vi "Dresden R2R Sputter 03.02.2018 IY24.vi"() -> ()   [LabVIEW 2009] (continued)
                        n624 = local read "Ch3_Bp_bv_open_L_safety"() -> (w1488)
                        n625 = case shown="False" w1488 {
                          frame #0 {
                            n626 = local write "Error Message"(data[5B] ("Error Message")) -> ()
                          }
                          frame #1 {
                            n627 = local write "Ch3_4_4_do"(T/1 ("Ch3_Do_Bp_bv_L")) -> ()
                          }
                        }
                      }
                    }
                    n628 = case shown="True" w1483 {
                      frame #0 {
                      }
                      frame #1 {
                        n629 = local read "Ch3_Bp_bv_close_L_safety"() -> (w1485)
                        n630 = case shown="False" w1485 {
                          frame #0 {
                            n631 = local write "Error Message"(data[5B] ("Error Message")) -> ()
                          }
                          frame #1 {
                            n632 = local write "Ch3_4_4_do"(i16? 0 ("Ch3_Do_Bp_bv_L")) -> ()
                          }
                        }
                      }
                    }
                  }
                }
                n633 = stacked-sequence {
                  frame #0 {
                    n634 = Or(x="Bp_bv_open_ch1_R_gui", y="Bp_bv_open_ch1_R") -> (x .or. y?=w1532)
                    n635 = Or(x="Bp_bv_close_ch1_R_gui", y="Bp_bv_close_ch1_R") -> (x .or. y?=w1531)
                    n636 = case shown="True" w1531 {
                      frame #0 {
                      }
                      frame #1 {
                        n637 = local read "Ch1_Bp_bv_close_R_safety"() -> (w1533)
                        n638 = case shown="True" w1533 {
                          frame #0 {
                            n639 = local write "Error Message"("BP-BV can not be opened.\nReason: SP does not work \nwhen system is under vacuum. \nIf system is  not under vacuum, TP-BV \nor PL-VBV  can be  open,or \nMP can work." ("Error Message")) -> ()
                          }
                          frame #1 {
                          }
                        }
                      }
                    }
                    n640 = case shown="True" w1532 {
                      frame #0 {
                      }
                      frame #1 {
                        n641 = local read "Ch1_Bp_bv_open_R_safety"() -> (w1535)
                        n642 = case shown="True" w1535 {
                          frame #0 {
                            n643 = local write "Error Message"("BP-BV can not be opened.\nReason: SP does not work \nwhen system is under vacuum. \nIf system is  not under vacuum, TP-BV \nor PL-VBV  can be  open,or \nMP can work." ("Error Message")) -> ()
                          }
                          frame #1 {
                          }
                        }
                      }
                    }
                  }
                }
                n644 = stacked-sequence {
                  frame #0 {
                    n645 = Or(x="Bp_bv_close_ch4_L_gui", y="Bp_bv_close_ch4_L") -> (x .or. y?=w1472)
                    n646 = Or(x="Bp_bv_open_ch4_L_gui", y="Bp_bv_open_ch4_L") -> (x .or. y?=w1467)
                    n647 = case shown="True" w1467 {
                      frame #0 {
                      }
                      frame #1 {
                        n648 = local read "Ch4_Bp_bv_open_L_safety"() -> (w1476)
                        n649 = case shown="True" w1476 {
                          frame #0 {
                            n650 = local write "Error Message"("BP-BV can not be opened.\nReason: SP does not work \nwhen system is under vacuum. \nIf system is  not under vacuum, TP-BV \nor PL-VBV  can be  open,or \nMP can work." ("Error Message")) -> ()
                          }
                          frame #1 {
                            n651 = local write "Ch4_4_4_do"(T/1 ("Ch3_Do_Bp_bv_L")) -> ()
                          }
                        }
                      }
                    }
                    n652 = case shown="True" w1472 {
                      frame #0 {
                      }
                      frame #1 {
                        n653 = local read "Ch4_Bp_bv_close_L_safety"() -> (w1473)
                        n654 = case shown="True" w1473 {
                          frame #0 {
                            n655 = local write "Error Message"("BP-BV can not be opened.\nReason: SP does not work \nwhen system is under vacuum. \nIf system is  not under vacuum, TP-BV \nor PL-VBV  can be  open,or \nMP can work." ("Error Message")) -> ()
                          }
                          frame #1 {
                            n656 = local write "Ch4_4_4_do"(i16? 0 ("Ch3_Do_Bp_bv_L")) -> ()
                          }
                        }
                      }
                    }
                  }
                }
                n657 = stacked-sequence {
                  frame #0 {
                    n658 = Or(x="Bp_bv_open_ch2_R_gui", y="Bp_bv_open_ch2_R") -> (x .or. y?=w1519)
                    n659 = Or(x="Bp_bv_close_ch2_R_gui", y="Bp_bv_close_ch2_R") -> (x .or. y?=w1520)
                    n660 = case shown="True" w1519 {
                      frame #0 {
                      }
                      frame #1 {
                        n661 = local read "Ch2_Bp_bv_open_R_safety"() -> (w1524)
                        n662 = case shown="True" w1524 {
                          frame #0 {
                            n663 = local write "Error Message"("BP-BV can not be opened.\nReason: SP does not work \nwhen system is under vacuum. \nIf system is  not under vacuum, TP-BV \nor PL-VBV  can be  open,or \nMP can work." ("Error Message")) -> ()
                          }
                          frame #1 {
                            n664 = local write "Ch2_4_3_do"(T/1 ("Ch1_Do_Bp_bv_R")) -> ()
                          }
                        }
                      }
                    }
                    n665 = case shown="True" w1520 {
                      frame #0 {
                      }
                      frame #1 {
                        n666 = local read "Ch2_Bp_bv_close_R_safety"() -> (w1521)
                        n667 = case shown="True" w1521 {
                          frame #0 {
                            n668 = local write "Error Message"("BP-BV can not be opened.\nReason: SP does not work \nwhen system is under vacuum. \nIf system is  not under vacuum, TP-BV \nor PL-VBV  can be  open,or \nMP can work." ("Error Message")) -> ()
                          }
                          frame #1 {
                            n669 = local write "Ch2_4_3_do"(i16? 0 ("Ch1_Do_Bp_bv_R")) -> ()
                          }
                        }
                      }
                    }
                  }
                }
                n670 = stacked-sequence {
                  frame #0 {
                    n671 = Or(x="Bp_bv_open_ch3_R_gui", y="Bp_bv_open_ch3_R") -> (x .or. y?=w1503)
                    n672 = Or(x="Bp_bv_close_ch3_R_gui", y="Bp_bv_close_ch3_R") -> (x .or. y?=w1506)
                    n673 = case shown="True" w1503 {
                      frame #0 {
                      }
                      frame #1 {
                        n674 = local read "Ch3_Bp_bv_open_R_safety"() -> (w1512)
                        n675 = case shown="True" w1512 {
                          frame #0 {
                            n676 = local write "Error Message"("BP-BV can not be opened.\nReason: SP does not work \nwhen system is under vacuum. \nIf system is  not under vacuum, TP-BV \nor PL-VBV  can be  open,or \nMP can work." ("Error Message")) -> ()
                          }
                          frame #1 {
                            n677 = local write "Ch3_4_3_do"(T/1 ("Ch1_Do_Bp_bv_R")) -> ()
                          }
                        }
                      }
                    }
                    n678 = case shown="True" w1506 {
                      frame #0 {
                      }
                      frame #1 {
                        n679 = local read "Ch3_Bp_bv_close_R_safety"() -> (w1509)
                        n680 = case shown="True" w1509 {
                          frame #0 {
                            n681 = local write "Error Message"("BP-BV can not be opened.\nReason: SP does not work \nwhen system is under vacuum. \nIf system is  not under vacuum, TP-BV \nor PL-VBV  can be  open,or \nMP can work." ("Error Message")) -> ()
                          }
                          frame #1 {
                            n682 = local write "Ch3_4_3_do"(i16? 0 ("Ch1_Do_Bp_bv_R")) -> ()
                          }
                        }
                      }
                    }
                  }
                }
                n683 = stacked-sequence {
                  frame #0 {
                    n684 = Or(x="Bp_bv_open_ch2_L_gui", y="Bp_bv_open_ch2_L_tab") -> (x .or. y?=w1494)
                    n685 = Or(x="Bp_bv_close_ch2_L_gui", y="Bp_bv_close_ch2_L") -> (x .or. y?=w1491)
                    n686 = case shown="True" w1494 {
                      frame #0 {
                      }
                      frame #1 {
                        n687 = local read "Ch2_Bp_bv_open_L_safety"() -> (w1500)
                        n688 = case shown="False" w1500 {
                          frame #0 {
                            n689 = local write "Error Message"("BP-BV can not be opened.\nReason: SP does not work \nwhen system is under vacuum. \nIf system is  not under vacuum, TP-BV \nor PL-VBV  can be  open,or \nMP can work." ("Error Message")) -> ()
                          }
                          frame #1 {
                            n690 = local write "Ch2_4_4_do"(T/1 ("Ch1_Do_Bp_bv_R")) -> ()
                          }
                        }
                      }
                    }
                    n691 = case shown="True" w1491 {
                      frame #0 {
                      }
                      frame #1 {
                        n692 = local read "Ch2_Bp_bv_close_L_safety"() -> (w1497)
                        n693 = case shown="False" w1497 {
                          frame #0 {
                            n694 = local write "Error Message"("BP-BV can not be opened.\nReason: SP does not work \nwhen system is under vacuum. \nIf system is  not under vacuum, TP-BV \nor PL-VBV  can be  open,or \nMP can work." ("Error Message")) -> ()
                          }
                          frame #1 {
                            n695 = local write "Ch2_4_4_do"(i16? 0 ("Ch1_Do_Bp_bv_R")) -> ()
                          }
                        }
                      }
                    }
                  }
                }
              }
              frame #1 {
              }
            }
          }
        }
        n696 = stacked-sequence {
          frame #0 {
            n697 = Or(x="Ch1_Ch_vbv_open_gui", y="Ch1_Ch_vbv_open") -> (x .or. y?=w1542)
            n698 = Or(x="Ch1_Ch_vbv_close_gui", y="Ch1_Ch_vbv_close") -> (x .or. y?=w1541)
            n699 = case shown="True" w1542 {
              frame #0 {
              }
              frame #1 {
                n700 = local read "Ch1_Ch_vbv_open_safety"() -> (w1562)
                n701 = case shown="False" w1562 {
                  frame #0 {
                    n702 = local write "Error Message"("CH-VBV can not be opened.\nReason : * TP-BV can be open.     \n *Tp can not be stopped.\n*CH-CC can be open.    \n*BG-BV can be open.     " ("Error Message")) -> ()
                  }
                  frame #1 {
                    n703 = stacked-sequence {
                      frame #0 {
                        n704 = local write "Ch1_Ch_atm_do"(i16? 0 ("Ch1_Ch_vbv_do")) -> ()
                      }
                      frame #1 {
                        n705 = Wait (ms)(milliseconds to wait=i32? 500) -> ()  [unwired: 1 out]
                      }
                      frame #2 {
                        n706 = local write "Ch1_Ch_vbv_do"(T/1 ("Ch1_Ch_vbv_do")) -> ()
                      }
                      frame #3 {
                        n707 = Wait (ms)(milliseconds to wait=i32? 500) -> ()  [unwired: 1 out]
                      }
                    }
                  }
                }
              }
            }
            n708 = case shown="True" w1541 {
              frame #0 {
              }
              frame #1 {
                n709 = local write "Ch1_Ch_vbv_do"(i16? 0 ("Ch1_Ch_vbv_do")) -> ()
              }
            }
            n710 = Or(x="Ch2_Ch_vbv_open_gui", y="Ch2_Ch_vbv_open") -> (x .or. y?=w1559)
            n711 = Or(x="Ch2_Ch_vbv_close", y="Ch2_Ch_vbv_close_gui") -> (x .or. y?=w1560)
            n712 = case shown="True" w1559 {
              frame #0 {
              }
              frame #1 {
                n713 = local read "Ch2_Ch_vbv_open_safety"() -> (w1583)
                n714 = case shown="False" w1583 {
                  frame #0 {
                    n715 = local write "Error Message"("CH-VBV can not be opened.\nReason : * TP-BV can be open.     \n *Tp can not be stopped.\n*CH-CC can be open.    \n*BG-BV can be open.     " ("Error Message")) -> ()
                  }
                  frame #1 {
                    n716 = stacked-sequence {
                      frame #0 {
                        n717 = local write "Ch2_Ch_atm_do"(i16? 0 ("Ch1_Ch_vbv_do")) -> ()
                      }
                      frame #1 {
                        n718 = Wait (ms)(milliseconds to wait=i32? 500) -> ()  [unwired: 1 out]
                      }
                      frame #2 {
                        n719 = local write "Ch2_Ch_vbv_do"(T/1 ("Ch1_Ch_vbv_do")) -> ()
                      }
                      frame #3 {
                        n720 = Wait (ms)(milliseconds to wait=i32? 500) -> ()  [unwired: 1 out]
                      }
                    }
                  }
                }
              }
            }
            n721 = case shown="False" w1560 {
              frame #0 {
              }
              frame #1 {
                n722 = local write "Ch2_Ch_vbv_do"(i16? 0 ("Ch1_Ch_vbv_do")) -> ()
              }
            }
            n723 = Or(x="Ch3_Ch_vbv_open_gui", y="Ch3_Ch_vbv_open") -> (x .or. y?=w1558)
            n724 = Or(x="Ch3_Ch_vbv_close_gui", y="Ch3_Ch_vbv_close") -> (x .or. y?=w1557)
            n725 = case shown="True" w1558 {
              frame #0 {
              }
              frame #1 {
                n726 = local read "Ch3_Ch_vbv_open_safety"() -> (w1576)
                n727 = case shown="True" w1576 {
                  frame #0 {
                    n728 = local write "Error Message"("CH-VBV can not be opened.\nReason : * TP-BV can be open.     \n *Tp can not be stopped.\n*CH-CC can be open.    \n*BG-BV can be open.     " ("Error Message")) -> ()
                  }
                  frame #1 {
                    n729 = stacked-sequence {
                      frame #0 {
                        n730 = local write "Ch3_Ch_atm_do"(i16? 0 ("Ch1_Ch_vbv_do")) -> ()
                      }
                      frame #1 {
                        n731 = Wait (ms)(milliseconds to wait=i32? 500) -> ()  [unwired: 1 out]
                      }
                      frame #2 {
                        n732 = local write "Ch3_Ch_vbv_do"(T/1 ("Ch1_Ch_vbv_do")) -> ()
                      }
                      frame #3 {
                        n733 = Wait (ms)(milliseconds to wait=i32? 500) -> ()  [unwired: 1 out]
                      }
                    }
                  }
                }
              }
            }
            n734 = case shown="True" w1557 {
              frame #0 {
              }
              frame #1 {
                n735 = local write "Ch3_Ch_vbv_do"(i16? 0 ("Ch1_Ch_vbv_do")) -> ()
              }
            }
            n736 = Or(x="Ch4_Ch_vbv_open_gui", y="Ch4_Ch_vbv_open") -> (x .or. y?=w1556)
            n737 = Or(x="Ch4_Ch_vbv_close_gui", y="Ch4_Ch_vbv_close") -> (x .or. y?=w1555)
            n738 = case shown="True" w1555 {
              frame #0 {
              }
              frame #1 {
                n739 = local write "Ch4_Ch_vbv_do"(i16? 0 ("Ch1_Ch_vbv_do")) -> ()
              }
            }
            n740 = case shown="True" w1556 {
              frame #0 {
              }
              frame #1 {
                n741 = local read "Ch4_Ch_vbv_open_safety"() -> (w1569)
                n742 = case shown="True" w1569 {
                  frame #0 {
                    n743 = local write "Error Message"("CH-VBV can not be opened.\nReason : * TP-BV can be open.     \n *Tp can not be stopped.\n*CH-CC can be open.    \n*BG-BV can be open.     " ("Error Message")) -> ()
                  }
                  frame #1 {
                    n744 = stacked-sequence {
                      frame #0 {
                        n745 = local write "Ch4_Ch_atm_do"(i16? 0 ("Ch1_Ch_vbv_do")) -> ()
                      }
                      frame #1 {
                        n746 = Wait (ms)(milliseconds to wait=i32? 500) -> ()  [unwired: 1 out]
                      }
                      frame #2 {
                        n747 = local write "Ch4_Ch_vbv_do"(T/1 ("Ch1_Ch_vbv_do")) -> ()
                      }
                      frame #3 {
                        n748 = Wait (ms)(milliseconds to wait=i32? 500) -> ()  [unwired: 1 out]
                      }
                    }
                  }
                }
              }
            }
          }
        }
        n749 = case shown="True" "MW1_off" {
          frame #0 {
          }
          frame #1 {
            n750 = flat-sequence {
              frame #0 {
                w1124 = data[3B] ("Ar_sccm3_4")
                n751 = local write "Microwave_Power"(w1124) -> ()
                n752 = local write "Ch1_MW1"(w1124) -> ()
              }
              frame #1 {
                n753 = Wait (ms)(milliseconds to wait=i32? 200) -> ()  [unwired: 1 out]
                n754 = local write "MW1_off"(i16? 0 ("MW1_off")) -> ()
              }
              frame #2 {
                n755 = local write "MW1_OPENED"(i16? 0 ("MW1_OPENED")) -> ()
                n756 = local write "Ch1_MW1_set"(T/1 ("Ch1_MW1_auto_set")) -> ()
              }
            }
          }
        }
        n757 = case shown="True" "MW2_off" {
          frame #0 {
          }
          frame #1 {
            n758 = flat-sequence {
              frame #0 {
                w1119 = data[3B] ("Ch1_MW2")
                n759 = local write "Microwave2_Power"(w1119) -> ()
                n760 = local write "Ch1_MW2"(w1119) -> ()
              }
              frame #1 {
                n761 = local write "MW2_off"(i16? 0 ("MW2_off")) -> ()
                n762 = Wait (ms)(milliseconds to wait=i32? 200) -> ()  [unwired: 1 out]
              }
              frame #2 {
                n763 = local write "MW2_OPENED"(i16? 0 ("MW2_OPENED")) -> ()
                n764 = local write "Ch1_MW2_set"(T/1 ("Ch1_MW2_auto_set")) -> ()
              }
            }
          }
        }
        n765 = case shown="True" "MW1_set" {
          frame #0 {
          }
          frame #1 {
            n766 = local read "MW1_OPENED"() -> (w1106)
            n767 = case shown="True" w1106 {
              frame #0 {
              }
              frame #1 {
                n768 = stacked-sequence {
                  frame #0 {
                    n769 = local read "Microwave_Power"() -> (w1107)
                    n770 = local write "Ch1_MW1"(w1107) -> ()
                  }
                  frame #1 {
                    n771 = local write "Ch1_MW1_set"(T/1 ("Mfc2_Ar _set")) -> ()
                  }
                }
              }
            }
          }
        }
        n772 = case shown="True" "MW2_set" {
          frame #0 {
          }
          frame #1 {
            n773 = local read "MW2_OPENED"() -> (w1103)
            n774 = case shown="True" w1103 {
              frame #0 {
              }
              frame #1 {
                n775 = stacked-sequence {
                  frame #0 {
                    n776 = local read "Microwave2_Power"() -> (w1104)
                    n777 = local write "Ch1_MW2"(w1104) -> ()
                  }
                  frame #1 {
                    n778 = local write "Ch1_MW2_set"(T/1 ("Mfc2_Ar _set")) -> ()
                  }
                }
              }
            }
          }
        }
        n779 = case shown="True" "MW1_Power_on" {
          frame #0 {
          }
          frame #1 {
            n780 = stacked-sequence {
              frame #0 {
                n781 = local write "Ch1_MW1"("Microwave_Power") -> ()
              }
              frame #1 {
                n782 = Wait (ms)(milliseconds to wait=i32? 200) -> ()  [unwired: 1 out]
              }
              frame #2 {
                n783 = local write "Ch1_MW1_set"(T/1 ("Ch1_MW1_set")) -> ()
              }
              frame #3 {
                n784 = Wait (ms)(milliseconds to wait=i32? 1000) -> ()  [unwired: 1 out]
                "MW1_OPENED" <- T/1 ("Open")
              }
            }
          }
        }
        n785 = case shown="True" "MW2_Power_ON" {
          frame #0 {
          }
          frame #1 {
            n786 = stacked-sequence {
              frame #0 {
                n787 = local write "Ch1_MW2"("Microwave2_Power") -> ()
              }
              frame #1 {
                n788 = Wait (ms)(milliseconds to wait=i32? 200) -> ()  [unwired: 1 out]
              }
              frame #2 {
                n789 = local write "Ch1_MW2_set"(T/1 ("Ch1_MW1_set")) -> ()
              }
              frame #3 {
                n790 = Wait (ms)(milliseconds to wait=i32? 1000) -> ()  [unwired: 1 out]
                "MW2_OPENED" <- T/1 ("Open")
              }
            }
          }
        }
        n791 = stacked-sequence {
          frame #0 {
            n792 = stacked-sequence {
              frame #0 {
                n793 = Or(x="Ch4_sov_Ar_top_open gui", y="Ch4_sov_Ar_top_open tab") -> (x .or. y?=w1290)
                n794 = Or(x="Ch4_sov_Ar_top_close tab", y="Ch4_sov_Ar_top_close gui") -> (x .or. y?=w1289)
                n795 = case shown="True" w1289 {
                  frame #0 {
                  }
                  frame #1 {
                    n796 = local read "Ch4_sov_Ar_close_safety"() -> (w1293)
                    n797 = case shown="True" w1293 {
                      frame #0 {
                        n798 = local write "Error Message"(data[5B] ("Error Message")) -> ()
                      }
                      frame #1 {
                        n799 = local write "Ch4_Sov_Ar_do"(i16? 0 ("Ch1_Sov_Ar_do")) -> ()
                      }
                    }
                  }
                }
                n800 = case shown="True" w1290 {
                  frame #0 {
                  }
                  frame #1 {
                    n801 = local read "Ch4_sov_Ar_open_safety"() -> (w1296)
                    n802 = case shown="True" w1296 {
                      frame #0 {
                        n803 = local write "Error Message"(data[5B] ("Error Message")) -> ()
                      }
                      frame #1 {
                        n804 = local write "Ch4_Sov_Ar_do"(T/1 ("Ch1_Sov_Ar_do")) -> ()
                      }
                    }
                  }
                }
              }
            }
            n805 = stacked-sequence {
              frame #0 {
                n806 = Or(x="Ch3_sov_Ar_top_open gui", y="Ch3_sov_Ar_top_open") -> (x .or. y?=w1280)
                n807 = Or(x="Ch3_sov_Ar_top_close  gui", y="Ch3_sov_Ar_top_close") -> (x .or. y?=w1279)
                n808 = case shown="True" w1280 {
                  frame #0 {
                  }
                  frame #1 {
                    n809 = local read "Ch3_sov_Ar_open_safety"() -> (w1284)
                    n810 = case shown="True" w1284 {
                      frame #0 {
                        n811 = local write "Error Message"(data[5B] ("Error Message")) -> ()
                      }
                      frame #1 {
                        n812 = local write "Ch3_Sov_Ar_do"(T/1 ("Ch1_Sov_Ar_do")) -> ()
                      }
                    }
                  }
                }
                n813 = case shown="True" w1279 {
                  frame #0 {
                  }
                  frame #1 {
                    n814 = local read "Ch3_sov_Ar_close_safety"() -> (w1281)
                    n815 = case shown="True" w1281 {
                      frame #0 {
                        n816 = local write "Error Message"(data[5B] ("Error Message")) -> ()
                      }
                      frame #1 {
                        n817 = local write "Ch3_Sov_Ar_do"(i16? 0 ("Ch1_Sov_Ar_do")) -> ()
                      }
                    }
                  }
                }
              }
            }
            n818 = stacked-sequence {
              frame #0 {
                n819 = Or(x="Ch1_sov_Ar_top_open_gui", y="Ch1_sov_Ar_top_open  tab") -> (x .or. y?=w1253)
                n820 = Or(x="Ch1_sov_Ar_top_close_gui", y="Ch1_sov_Ar_top_close  tab") -> (x .or. y?=w1256)
                n821 = case shown="True" w1253 {
                  frame #0 {
                  }
                  frame #1 {
                    n822 = local read "Ch1_sov_Ar_open_safety"() -> (w1260)
                    n823 = case shown="True" w1260 {
                      frame #0 {
                        n824 = local write "Error Message"(data[5B] ("Error Message")) -> ()
                      }
                      frame #1 {
                        n825 = local write "Ch1_Sov_Ar_do"(T/1 ("Ch1_Sov_Ar_do")) -> ()
                      }
                    }
                  }
                }
                n826 = case shown="True" w1256 {
                  frame #0 {
                  }
                  frame #1 {
                    n827 = local read "Ch1_sov_Ar_close_safety"() -> (w1257)
                    n828 = case shown="True" w1257 {
                      frame #0 {
                        n829 = local write "Error Message"(data[5B] ("Error Message")) -> ()
                      }
                      frame #1 {
                        n830 = local write "Ch1_Sov_Ar_do"(i16? 0 ("Ch1_Sov_Ar_do")) -> ()
                      }
                    }
                  }
                }
              }
            }
            n831 = stacked-sequence {
              frame #0 {
                n832 = Or(x="Ch2_sov_Ar_front_open gui", y="Ch2_sov_Ar_front_open  tab") -> (x .or. y?=w1268)
                n833 = Or(x="Ch2_sov_Ar_top_close  gui", y="Ch2_sov_Ar_top_close  tab") -> (x .or. y?=w1267)
                n834 = case shown="True" w1268 {
                  frame #0 {
                  }
                  frame #1 {
                    n835 = local read "Ch2_sov_Ar_open_safety"() -> (w1272)
                    n836 = case shown="True" w1272 {
                      frame #0 {
                        n837 = local write "Error Message"(data[5B] ("Error Message")) -> ()
                      }
                      frame #1 {
                        n838 = local write "Ch2_Sov_Ar_do"(T/1 ("Ch1_Sov_Ar_do")) -> ()
                      }
                    }
                  }
                }
                n839 = case shown="True" w1267 {
                  frame #0 {
                  }
                  frame #1 {
                    n840 = local read "Ch2_sov_Ar_close_safety"() -> (w1269)
                    n841 = case shown="True" w1269 {
                      frame #0 {
                        n842 = local write "Error Message"(data[5B] ("Error Message")) -> ()
                      }
                      frame #1 {
                        n843 = local write "Ch2_Sov_Ar_do"(i16? 0 ("Ch1_Sov_Ar_do")) -> ()
                      }
                    }
                  }
                }
              }
            }
          }
        }
        n844 = stacked-sequence {
          frame #0 {
            n845 = case shown="True" "Ch2_dc_active" {
              frame #0 {
              }
              frame #1 {
                w992 = i16? 0 ("Ch2_dc_active")
                w993 = i16? 0 ("Cnt_Dcps_sw2_do")
                w994 = T/1 ("Cnt_Dcps_sw1_do")
                n846 = local write "Cnt_Dcps_sw1_do"(w994) -> ()
                n847 = local write "Ch2_WFC_do"(w994) -> ()
                n848 = local write "Ch3_dc_active"(w992) -> ()
                n849 = local write "Ch4_rf_active"(w992) -> ()
                n850 = local write "Ch1_mw_active"(w992) -> ()
                n851 = local write "Cnt_Dcps_sw2_do"(w993) -> ()
                n852 = local write "Ch1_WFC_do"(w993) -> ()
                n853 = local write "Ch3_WFC_do"(w993) -> ()
                n854 = local write "Ch4_WFC_do"(w993) -> ()
              }
            }
            n855 = case shown="True" "Ch3_dc_active" {
              frame #0 {
              }
              frame #1 {
                w989 = i16? 0 ("Ch2_dc_active")
                w990 = i16? 0 ("Cnt_Dcps_sw2_do")
                w991 = T/1 ("Cnt_Dcps_sw1_do")
                n856 = local write "Cnt_Dcps_sw2_do"(w991) -> ()
                n857 = local write "Ch3_WFC_do"(w991) -> ()
                n858 = local write "Ch2_dc_active"(w989) -> ()
                n859 = local write "Ch4_rf_active"(w989) -> ()
                n860 = local write "Ch1_mw_active"(w989) -> ()
                n861 = local write "Cnt_Dcps_sw1_do"(w990) -> ()
                n862 = local write "Ch1_WFC_do"(w990) -> ()
                n863 = local write "Ch2_WFC_do"(w990) -> ()
                n864 = local write "Ch4_WFC_do"(w990) -> ()
              }
            }
            n865 = case shown="True" "Ch4_rf_active" {
              frame #0 {
              }
              frame #1 {
                w986 = i16? 0 ("Ch2_dc_active")
                w987 = i16? 0 ("Cnt_Dcps_sw2_do")
                n866 = local write "Ch4_WFC_do"(T/1 ("Cnt_Dcps_sw1_do")) -> ()
                n867 = local write "Ch2_dc_active"(w986) -> ()
                n868 = local write "Ch3_dc_active"(w986) -> ()
                n869 = local write "Ch1_mw_active"(w986) -> ()
                n870 = local write "Ch1_WFC_do"(w987) -> ()
                n871 = local write "Ch3_WFC_do"(w987) -> ()
                n872 = local write "Ch2_WFC_do"(w987) -> ()
              }
            }
            n873 = case shown="True" "Ch1_mw_active" {
              frame #0 {
              }
              frame #1 {
                w983 = i16? 0 ("Ch2_dc_active")
                w984 = i16? 0 ("Cnt_Dcps_sw2_do")
                n874 = local write "Ch3_dc_active"(w983) -> ()
                n875 = local write "Ch4_rf_active"(w983) -> ()
                n876 = local write "Ch1_WFC_do"(T/1 ("Cnt_Dcps_sw1_do")) -> ()
                n877 = local write "Ch2_dc_active"(w983) -> ()
                n878 = local write "Ch3_WFC_do"(w984) -> ()
                n879 = local write "Ch2_WFC_do"(w984) -> ()
                n880 = local write "Ch4_WFC_do"(w984) -> ()
              }
            }
          }
        }
        n881 = stacked-sequence {
          frame #0 {
            n882 = stacked-sequence {
              frame #0 {
                n883 = Compound Arithmetic op=OR("Ch2_Cc_close_tab gui", "Ch2_Cc_close_tab", "Ch2_Cc_close_top gui", "Ch2_Cc_close_top") -> (w1227)
                n884 = Compound Arithmetic op=OR("Ch2_Cc_open_tab_gui", "Ch2_Cc_open_tab", "Ch2_Cc_open_top gui", "Ch2_Cc_open_top") -> (w1230)
                n885 = case shown="True" w1230 {
                  frame #0 {
                  }
                  frame #1 {
                    n886 = local read "Ch2_Cc_open_safety"() -> (w1234)
                    n887 = case shown="True" w1234 {
                      frame #0 {
                        n888 = local write "Error Message"("CH-CC can not be opened.\nReason :* CH pressure is not suitable. \n*Tp can not be stopped.        \n*There is gas flow.                  " ("Error Message")) -> ()
                      }
                      frame #1 {
                        n889 = local write "Ch2_Cc_on_off_do"(T/1 ("Ch1_Ch_cc_on_off_do")) -> ()
                      }
                    }
                  }
                }
                n890 = case shown="True" w1227 {
                  frame #0 {
                  }
                  frame #1 {
                    n891 = local write "Ch2_Cc_on_off_do"(i16? 0 ("Ch1_Ch_cc_on_off_do")) -> ()
                  }
                }
              }
            }
            n892 = stacked-sequence {
              frame #0 {
                n893 = Compound Arithmetic op=OR("Ch4_Cc_close_tab_gui", "Ch4_Cc_close_tab", "Ch4_Cc_top_close_gui", "Ch4_CC_top_close") -> (w1204)
                n894 = Compound Arithmetic op=OR("Ch4_Cc_open_tab_gui", "Ch4_Cc_open_tab", "Ch4_Cc_top_open_gui", "Ch4_Cc_top_open") -> (w1201)
                n895 = case shown="True" w1201 {
                  frame #0 {
                  }
                  frame #1 {
                    n896 = local read "Ch4_Cc_open_safety"() -> (w1206)
                    n897 = case shown="True" w1206 {
                      frame #0 {
                        n898 = local write "Error Message"("CH-CC can not be opened.\nReason :* CH pressure is not suitable.\n*Tp can not be stopped.       \n*There is gas flow.                 " ("Error Message")) -> ()
                      }
                      frame #1 {
                        n899 = local write "Ch4_Cc_on_off_do"(T/1 ("Ch1_Ch_cc_on_off_do")) -> ()
                      }
                    }
                  }
                }
                n900 = case shown="True" w1204 {
                  frame #0 {
                  }
                  frame #1 {
                    n901 = local write "Ch4_Cc_on_off_do"(i16? 0 ("Ch1_Ch_cc_on_off_do")) -> ()
                  }
                }
              }
            }
            n902 = stacked-sequence {
              frame #0 {
                n903 = Compound Arithmetic op=OR("Ch1_Cc_open_tab_gui", "Ch1_Cc_open_tab", "Ch1_cc_open_top", "Ch1_cc_open_top gui") -> (w1244)
                n904 = Compound Arithmetic op=OR("Ch1_Cc_close_tab_gui", "Ch1_Cc_close_tab", "Ch1_Cc_close_top", "Ch1_Cc_close_top gui") -> (w1243)
                n905 = case shown="True" w1244 {
                  frame #0 {
                  }
                  frame #1 {
                    n906 = local read "Ch1_Cc_open_safety"() -> (w1248)
                    n907 = case shown="True" w1248 {
                      frame #0 {
                        n908 = local write "Error Message"("CH-CC can not be opened.\nReason :* CH pressure is not suitable. \n*Tp can not be stopped.        \n*There is gas flow.                  " ("Error Message")) -> ()
                      }
                      frame #1 {
                        n909 = local write "Ch1_Cc_on_off_do"(T/1 ("Ch1_Ch_cc_on_off_do")) -> ()
                      }
                    }
                  }
                }
                n910 = case shown="True" w1243 {
                  frame #0 {
                  }
                  frame #1 {
                    n911 = local write "Ch1_Cc_on_off_do"(i16? 0 ("Ch1_Ch_cc_on_off_do")) -> ()
                  }
                }
              }
            }
            n912 = stacked-sequence {
              frame #0 {
                n913 = Compound Arithmetic op=OR("Ch3_Cc_close_tab_gui", "Ch3_Cc_close_tab", "Ch3_Cc_top_close gui", "Ch3_Cc_top_close") -> (w1213)
                n914 = Compound Arithmetic op=OR("Ch3_Cc_open_tab gui", "Ch3_Cc_open_tab", "Ch3_Cc_top_open_gui", "Ch3_Cc_top_open") -> (w1216)
                n915 = case shown="True" w1216 {
                  frame #0 {
                  }
                  frame #1 {
                    n916 = local read "Ch3_Cc_open_safety"() -> (w1220)
                    n917 = case shown="True" w1220 {
                      frame #0 {
                        n918 = local write "Error Message"("CH-CC can not be opened.\nReason :* CH pressure is not suitable.\n*Tp can not be stopped.       \n*There is gas flow.                 " ("Error Message")) -> ()
                      }
                      frame #1 {
                        n919 = local write "Ch3_Cc_on_off_do"(T/1 ("Ch1_Ch_cc_on_off_do")) -> ()
                      }
                    }
                  }
                }
                n920 = case shown="True" w1213 {
                  frame #0 {
                  }
                  frame #1 {
                    n921 = local write "Ch3_Cc_on_off_do"(i16? 0 ("Ch1_Ch_cc_on_off_do")) -> ()
                  }
                }
              }
            }
          }
        }
        n922 = stacked-sequence {
          frame #0 {
            w1053 = i32? 1 ("x")
            w1052 = i32? 99 ("x")
            n923 = local read "Pc_bv1_position"() -> (w1051)
            n924 = In Range and Coerce(upper limit=w1052, x=w1051, lower limit=w1053) -> (In Range?=w1054)  [unwired: 1 out]
            n925 = Greater Or Equal?(x=w1051, y=w1052) -> (x >= y?=w1056)
            n926 = Less Or Equal?(x=w1051, y=w1053) -> (x <= y?=w1055)
            n927 = case shown="True" w1056 {
              frame #0 {
              }
              frame #1 {
                w1061 = T/1 ("Pc_bv_on(ch1)")
                n928 = local write "Ch1_Pc_bv_on"(w1061) -> ()
                n929 = local write "Ch1_Pc_bv_middle"(i16? 0 ("Pc_bv_middle(ch1)")) -> ()
                "Pc_bv_opened_ch1" <- w1061
              }
            }
            n930 = case shown="True" w1055 {
              frame #0 {
              }
              frame #1 {
                w1060 = i16? 0 ("Pc_bv_on(ch1)")
                n931 = local write "Ch1_Pc_bv_middle"(w1060) -> ()
                n932 = local write "Ch1_Pc_bv_on"(w1060) -> ()
                "Pc_bv_closed_ch1" <- T/1 ("Pc_bv_closed")
              }
            }
            n933 = case shown="True" w1054 {
              frame #0 {
              }
              frame #1 {
                n934 = local write "Ch1_Pc_bv_on"(i16? 0 ("Pc_bv_on(ch1)")) -> ()
                n935 = local write "Ch1_Pc_bv_middle"(T/1 ("Pc_bv_middle(ch1)")) -> ()
              }
            }
          }
          frame #1 {
            n936 = Wait (ms)(milliseconds to wait=i32? 10) -> ()  [unwired: 1 out]
          }
          frame #2 {
            w1064 = i32? 1 ("x")
            w1066 = i32? 99 ("x")
            n937 = local read "Pc_bv2_position"() -> (w1065)
            n938 = Greater Or Equal?(x=w1065, y=w1066) -> (x >= y?=w1069)
            n939 = In Range and Coerce(upper limit=w1066, x=w1065, lower limit=w1064) -> (In Range?=w1067)  [unwired: 1 out]
            n940 = Less Or Equal?(x=w1065, y=w1064) -> (x <= y?=w1068)
            n941 = case shown="True" w1069 {
              frame #0 {
              }
              frame #1 {
                w1074 = T/1 ("Pc_bv_on(ch1)")
                n942 = local write "Ch2_Pc_bv_on"(w1074) -> ()
                n943 = local write "Ch2_Pc_bv_middle"(i16? 0 ("Pc_bv_middle(ch1)")) -> ()
                "Pc_bv_opened_ch2" <- w1074
              }
            }
            n944 = case shown="True" w1068 {
              frame #0 {
              }
              frame #1 {
                w1073 = i16? 0 ("Pc_bv_on(ch1)")
                n945 = local write "Ch2_Pc_bv_on"(w1073) -> ()
                n946 = local write "Ch2_Pc_bv_middle"(w1073) -> ()
                "Pc_bv_closed_ch2" <- T/1 ("Pc_bv_closed_ch2")
              }
            }
            n947 = case shown="True" w1067 {
              frame #0 {
              }
              frame #1 {
                n948 = local write "Ch2_Pc_bv_on"(i16? 0 ("Pc_bv_on(ch1)")) -> ()
                n949 = local write "Ch2_Pc_bv_middle"(T/1 ("Pc_bv_middle(ch1)")) -> ()
              }
            }
          }
          frame #3 {
            n950 = Wait (ms)(milliseconds to wait=i32? 10) -> ()  [unwired: 1 out]
          }
          frame #4 {
            w1077 = i32? 1 ("x")
            w1079 = i32? 99 ("x")
            n951 = local read "Pc_bv3_position"() -> (w1078)
            n952 = In Range and Coerce(upper limit=w1079, x=w1078, lower limit=w1077) -> (In Range?=w1080)  [unwired: 1 out]
            n953 = Greater Or Equal?(x=w1078, y=w1079) -> (x >= y?=w1082)
            n954 = Less Or Equal?(x=w1078, y=w1077) -> (x <= y?=w1081)
            n955 = case shown="True" w1082 {
              frame #0 {
              }
              frame #1 {
                w1087 = T/1 ("Pc_bv_on(ch1)")
                n956 = local write "Ch3_Pc_bv_on"(w1087) -> ()
                n957 = local write "Ch3_Pc_bv_middle"(i16? 0 ("Pc_bv_middle(ch1)")) -> ()
                "Pc_bv_opened_ch3" <- w1087
              }
            }
            n958 = case shown="True" w1081 {
              frame #0 {
              }
              frame #1 {
                w1086 = i16? 0 ("Pc_bv_on(ch1)")
                n959 = local write "Ch3_Pc_bv_on"(w1086) -> ()
                n960 = local write "Ch3_Pc_bv_middle"(w1086) -> ()
                "Pc_bv_closed_ch3" <- T/1 ("Pc_bv_closed_ch3")
              }
            }
            n961 = case shown="True" w1080 {
              frame #0 {
              }
              frame #1 {
                n962 = local write "Ch3_Pc_bv_on"(i16? 0 ("Pc_bv_on(ch1)")) -> ()
                n963 = local write "Ch3_Pc_bv_middle"(T/1 ("Pc_bv_middle(ch1)")) -> ()
              }
            }
          }
          frame #5 {
            n964 = Wait (ms)(milliseconds to wait=i32? 10) -> ()  [unwired: 1 out]
          }
          frame #6 {
            w1090 = i32? 1 ("x")
            w1092 = i32? 99 ("x")
            n965 = local read "Pc_bv4_position"() -> (w1091)
            n966 = In Range and Coerce(upper limit=w1092, x=w1091, lower limit=w1090) -> (In Range?=w1093)  [unwired: 1 out]
            n967 = Greater Or Equal?(x=w1091, y=w1092) -> (x >= y?=w1095)
            n968 = Less Or Equal?(x=w1091, y=w1090) -> (x <= y?=w1094)
            n969 = case shown="True" w1095 {
              frame #0 {
              }
              frame #1 {
                w1100 = T/1 ("Pc_bv_on(ch1)")
                n970 = local write "Ch4_Pc_bv_on"(w1100) -> ()
                n971 = local write "Ch4_Pc_bv_middle"(i16? 0 ("Pc_bv_middle(ch1)")) -> ()
                "Pc_bv_opened_ch4" <- w1100
              }
            }
            n972 = case shown="True" w1094 {
              frame #0 {
              }
              frame #1 {
                w1099 = i16? 0 ("Pc_bv_on(ch1)")
                n973 = local write "Ch4_Pc_bv_on"(w1099) -> ()
                n974 = local write "Ch4_Pc_bv_middle"(w1099) -> ()
                "Pc_bv_closed_ch4" <- T/1 ("Pc_bv_closed_ch4")
              }
            }
            n975 = case shown="True" w1093 {
              frame #0 {
              }
              frame #1 {
                n976 = local write "Ch4_Pc_bv_on"(i16? 0 ("Pc_bv_on(ch1)")) -> ()
                n977 = local write "Ch4_Pc_bv_middle"(T/1 ("Pc_bv_middle(ch1)")) -> ()
              }
            }
          }
          frame #7 {
            n978 = Wait (ms)(milliseconds to wait=i32? 10) -> ()  [unwired: 1 out]
          }
        }
        n979 = stacked-sequence {
          frame #0 {
            # "Direction of Casette"
            n980 = local read "Counter_read_data"() -> (w999)
            n981 = feedback #6() -> (w1019)  [unwired: 1 in]
            n982 = In Range and Coerce(upper limit=i16? 2205, x=w999, lower limit=i16? 2155) -> (In Range?=w998)  [unwired: 1 out]
            n983 = In Range and Coerce(upper limit=i16? 6585, x=w999, lower limit=i16? 6535) -> (In Range?=w996)  [unwired: 1 out]
            n984 = In Range and Coerce(upper limit=i16? 25, x=w999, lower limit=i16? -25) -> (In Range?=w1008)  [unwired: 1 out]
            n985 = In Range and Coerce(upper limit=i16? 4380, x=w999, lower limit=i16? 4330) -> (In Range?=w997)  [unwired: 1 out]
            n986 = Greater?(x=w999, y=w1019) -> (0:w1017)
            n987 = Less?(x=w999, y=w1019) -> (x < y?=w1018)
            n988 = Build Array(i16? 0 ("element"), w1008, w998, w997, w996) -> (w1011)
            n989 = Boolean Array To Number(Boolean array=w1011) -> (number=w1010)
            n990 = Build Array(i16? 0 ("element"), w1017, w1018) -> (w1014)
            n991 = Mantissa & Exponent(0:w1010) -> (2:w995)  [unwired: 1 out]
            n992 = Boolean Array To Number(Boolean array=w1014) -> (number=w1015)
            n993 = case shown="1" w995 {
              frame #0 {
              }
              frame #1 {
                n994 = local write "ch_present_position"(dbl? 1.0 ("ch_present_position")) -> ()